vi "UHR-Fleezers Control (host) - 12.4.vi"() -> ()   [LabVIEW 2012] (continued)
          }
          frame #3 {
            n1108 = Wait (ms)(milliseconds to wait=u32 500) -> ()  [unwired: 1 out]
          }
          frame #4 {
            n1109 = property on="Confocal Image" class="Bool (strict)"("Val(Sgnl)"=TRUE ("Value (Signaling)")) -> ()  [unwired: 2 in, 2 out]
          }
          frame #5 {
            n1110 = Wait (ms)(milliseconds to wait=u32 2000) -> ()  [unwired: 1 out]
          }
          frame #6 {
            n1111 = while {
              stop <- w1611 stop-if-true
              n1112 = local read "Saving..."() -> (w1612:bool)
              n1113 = Not(x=w1612) -> (.not. x?=w1611:bool)
            }
          }
          frame #7 {
            n1114 = property on="Flip Green Filter" class="Bool (strict)"("Val(Sgnl)"=TRUE ("Value (Signaling)")) -> ()  [unwired: 2 in, 2 out]
            n1115 = property on="Green Laser ON" class="Bool (strict)"("Val(Sgnl)"=w1616) -> ()  [unwired: 2 in, 2 out]
            n1116 = property on="Laser interlacing mode" class="RadioBtnsControl (strict)"("Val(Sgnl)"=w1615) -> ()  [unwired: 2 in, 2 out]
          }
          frame #8 {
            n1117 = property on="Green FB On/Off" class="Bool (strict)"("Val(Sgnl)"=w1617) -> ()  [unwired: 2 in, 2 out]
          }
        }
      }
      event "Stop All": Value Change {
        n1118 = event-data() -> ()  [unwired: 1 in, 5 out]
        n1119 = local read "Delay (ms)"() -> (w1620:i32)
        n1120 = call "serial write macro.vi"("String"="l0", "Delay (ms)"=w1620, "VISA resource name"=w1623) -> ("read buffer"=w1618:string, "error out"=w1619:errorcluster, "VISA resource name out"=w1622:refnum<visa-resource-name>)
        n1121 = local write "read blue buffer"(w1618) -> ()
        n1122 = local write "Blue Error Out"(w1619) -> ()
        n1123 = VISA Close(VISA resource name=w1622) -> ()  [unwired: 1 in, 1 out]
        n1124 = local read "Stop All"() -> (w1624:bool)
      }
    }
    n1125 = node-c288() -> ()  [unwired: 1 in, 1 out]
  }
  n1126 = timed-loop "Basic control parameters (all FPGA settings, other basic controls)" {
    tunnel: w13 -> [w1633]
    shift-right: [w1632] -> _
    shift-left: errorcluster {"status"=FALSE, "code"=0, "source"=""} ("error out") -> [w1631]
    tunnel: [w1630] -> _
    timing: w127 -> [_]
    timing-out: [_] -> w126
    tunnel: w100 -> [w1629]
    tunnel: w72 -> [w1628]
    tunnel: w71 -> [w1627]
    tunnel: w70 -> [w1626]
    tunnel: w69 -> [w1625]
    stop <- w1630 stop-if-true
    n1127 = node-c288() -> ()  [unwired: 2 out]
    n1128 = event shown="[26] \"Invert APD Gate\", \"APD Gate ON Count\", \"APD Gate OFF Count\", \"APD Gate\", \"APD Integration Time (s)\", \"APD AO Scale Factor\", \"Duty Frequency (ON 1/N cycles)\", \"Interlace ON count\", \"Interlace OFF count\": Value Change" {
      selector: _ -> [_ _ _ _ _ _ _ _ _ _ _ _ _ _ _ _ _ _ _ _ _ _ _ _ _ _ _ _ _ _ _ _ _ _ _ _ _ _ _ _ _ _ _ _ _ _ _ _ _ _ _ _ _ _ _ _ _ _ _ _ _ _ _ _ _ _ _ _ _ _ _ _ _ _]
      dyn-events: _ -> [_ _ _ _ _ _ _ _ _ _ _ _ _ _ _ _ _ _ _ _ _ _ _ _ _ _ _ _ _ _ _ _ _ _ _ _ _ _ _ _ _ _ _ _ _ _ _ _ _ _ _ _ _ _ _ _ _ _ _ _ _ _ _ _ _ _ _ _ _ _ _ _ _ _]
      timeout: _ -> [_ _ _ _ _ _ _ _ _ _ _ _ _ _ _ _ _ _ _ _ _ _ _ _ _ _ _ _ _ _ _ _ _ _ _ _ _ _ _ _ _ _ _ _ _ _ _ _ _ _ _ _ _ _ _ _ _ _ _ _ _ _ _ _ _ _ _ _ _ _ _ _ _ _]
      tunnel: w1633 -> [w1674 _ _ _ w1712 _ w1734 _ _ _ _ w1800 _ _ w1843 w1849 w1856 w1861 w1952 _ w1968 w1993 w2014 w2035 w2056 w2085 w2111 w2114 w2118 w2213 w2218 w2256 _ w2291 w2295 w2306 w2310 w2314 _ w2322 _ _ _ _ _ _ _ _ _ _ _ _ _ _ _ _ _ w2700 _ w2717 _ w2724 w2742 _ w2749 w2757 w2772 w2788 w2794 _ w2803 _ w2822 _]
      tunnel: [w1673 _ _ _ w1702 _ w1733 _ _ w1765 _ w1779 _ _ w1842 w1845 w1855 w1858 w1946 _ w1967 w1992 w2012 w2033 w2054 w2079 w2109 _ w2116 w2211 w2216 w2254 _ w2289 w2293 w2297 w2308 w2312 _ w2320 _ _ _ _ _ _ _ _ _ _ _ _ _ _ _ _ _ w2698 _ _ _ _ w2739 _ _ _ _ _ _ _ _ _ _ _] -> w1632
      tunnel: w1631 -> [w1672 _ _ _ w1711 _ w1732 _ _ w1765 _ w1799 _ _ w1841 w1844 w1854 w1857 w1951 _ w1966 w1991 w2013 w2034 w2055 w2084 w2110 w2113 w2117 w2212 w2217 w2255 _ w2290 w2294 w2305 w2309 w2313 _ w2321 _ _ _ _ _ _ _ _ _ _ _ _ _ _ _ _ _ w2699 _ w2716 _ w2723 w2741 _ w2748 w2756 w2771 w2787 w2793 _ w2802 _ w2821 _]
      tunnel: [_ _ _ _ _ _ _ _ _ w1764 _ _ _ _ _ _ _ _ _ _ _ _ _ _ _ _ _ _ _ _ _ _ _ _ _ _ _ _ _ _ _ _ _ _ _ _ _ _ _ _ _ _ _ _ _ _ _ _ _ _ _ _ _ _ _ _ _ _ _ _ _ _ _ _] -> w1630
      tunnel: [_ _ _ _ _ _ _ "Round T1 X" _ _ _ _ _ _ _ _ _ _ _ _ _ _ _ _ _ _ _ _ _ _ _ _ _ _ _ _ _ _ _ _ _ _ _ _ _ _ _ _ _ _ _ _ _ _ _ _ _ _ _ _ _ _ _ _ _ _ _ _ _ _ _ _ _ _] -> _
      tunnel: [_ _ _ "Adjust Scale\nto Mean" _ _ _ _ _ _ _ _ _ _ _ _ _ _ _ _ _ _ _ _ _ _ _ _ "Test ttrig" _ _ _ _ _ _ _ _ _ _ _ _ _ _ _ _ _ _ "Flush Sample" "Flush Pump 3" "Flush Pump 1" "Clear Volume" _ _ _ _ _ _ _ _ _ _ _ _ _ _ _ _ _ _ _ _ _ _ _] -> _
      tunnel: [_ _ _ _ _ _ _ _ "Round T2 X" _ "Delayed Interlace Start" _ _ _ _ _ _ _ _ _ _ _ _ _ _ _ _ _ _ _ _ _ _ _ _ _ _ _ _ _ _ _ _ _ _ _ _ _ _ _ _ _ _ _ _ _ _ _ _ _ _ _ _ _ _ _ _ _ _ _ _ _ _ _] -> _
      tunnel: w1629 -> [_ _ _ _ _ _ _ _ _ _ _ _ _ _ _ _ _ _ _ _ _ _ _ _ _ _ _ _ _ _ _ _ _ _ _ _ _ _ _ _ _ _ _ w2479 w2486 w2493 w2498 w2507 _ _ w2613 _ _ _ _ _ _ _ _ _ _ _ _ _ _ _ _ _ _ _ _ _ _ _]
      tunnel: w1628 -> [_ _ _ _ _ _ _ _ _ _ _ _ _ _ _ _ _ _ _ _ _ _ _ _ _ _ _ _ _ _ _ _ _ _ _ _ _ _ _ _ _ w2396 _ _ _ _ _ _ w2551 _ _ w2619 _ w2628 _ w2642 _ _ _ _ _ _ _ _ _ _ _ _ _ _ _ _ _ _]
      tunnel: w1627 -> [_ _ _ _ _ _ _ _ _ _ _ _ _ _ _ _ _ _ _ _ _ _ _ _ _ _ _ _ _ _ _ _ _ _ _ _ _ _ _ _ _ _ _ _ _ _ _ _ _ _ _ _ _ _ _ _ _ _ _ _ _ _ _ _ _ _ _ _ _ _ _ _ _ _]
      tunnel: w1626 -> [_ _ _ _ _ _ _ _ _ _ _ _ _ _ _ _ _ _ _ _ _ _ _ _ _ _ _ _ _ _ _ _ _ _ _ _ _ _ _ _ w2333 _ _ _ _ _ _ _ _ w2581 _ _ w2624 _ w2635 _ w2667 _ _ _ _ _ _ _ _ _ _ _ _ _ _ _ _ _]
      tunnel: w1625 -> [_ _ _ _ _ _ _ _ _ _ _ _ _ _ _ _ _ _ _ _ _ _ _ _ _ _ _ _ _ _ _ _ _ _ _ _ _ _ _ _ _ _ _ _ _ _ _ _ _ _ _ _ _ _ _ _ _ _ _ _ _ _ _ _ _ _ _ _ _ _ _ _ _ _]
      event "AI Count (ticks)", "Sets to FIFO (Traps)", "Save ave N", "FPGA Ave.", "# Samples/channel", "N sets to save": Value Change {
        # "So that if 'Save ave N' is updated, the AOD scanning code updates too."
        n1129 = event-data() -> ()  [unwired: 6 out]
        n1130 = local read "AI Count (ticks)"() -> (w1656:u16)
        n1131 = Unbundle By Name("Sets to FIFO (Traps)") -> ("Set 1"=w1639:bool, "Set 2"=w1638:bool, "Set 3"=w1637:bool)
        n1132 = Boolean To (0,1)(Boolean="Sets to FIFO (Traps)") -> (0, 1=w1664:cluster{"Set 1":i16, "Set 2":i16, "Set 3":i16})
        n1133 = xnode "Read/Write Control"("FPGA VI Reference In"=w1674, "error in"=w1672, "ai count"=w1656, "Set 1"=w1639, "Set 2"=w1638, "Set 3"=w1637, "N of AI1 Int Acq Sets"="N Acq Sets (Traps + Fl.)") -> ("error out"=w1673:errorcluster)  [unwired: 1 out]
        n1134 = Cluster To Array(cluster=w1664) -> (array=w1663:i16[])
        n1135 = To Unsigned Long Integer(number=w1663) -> (unsigned 32bit integer=w1645:u32[])
        n1136 = local read "Scan steps (AOD)"() -> (w1665:u64)
        n1137 = Multiply(x=w1656, y="N Acq Sets (Traps + Fl.)") -> (x*y=w1654:u16)
        n1138 = Divide(x=40000000.0, y=w1656) -> (x/y=w1648:dbl)
        "AI rate (Hz)" <- w1648
        "Ave. Rate (Hz)" <- w1648
        n1139 = Add Array Elements(numeric array=w1645) -> (sum=w1657:u32)
        "Trap Sets" <- w1657
        n1140 = Reciprocal(x=w1648) -> (1/x=→"Ave. Period (s)":dbl)
        n1141 = property on="Scan steps (AOD)" class="DigNum (strict)"("Val(Sgnl)"=w1665) -> ()  [unwired: 2 in, 2 out]
        n1142 = Divide(x=w1648, y="N Acq Sets (Traps + Fl.)") -> (x/y=w1669:dbl)
        "Data Rate (Hz)" <- w1669
        n1143 = Reciprocal(x=w1669) -> (1/x=→"Data Period (s)":dbl)
        n1144 = local read "Save ave N"() -> (w1668:dbl)
        n1145 = Divide(x=w1669, y=w1668) -> (x/y=w1667:dbl)
        "Save Data Rate (Hz)" <- w1667
        n1146 = Reciprocal(x=w1667) -> (1/x=→"Save Data Period (s)":dbl)
        n1147 = Multiply(x=w1654, y="# Samples/trap") -> (x*y=w1652:u32)
        "Counts/DMA" <- w1652
        n1148 = property on="Trap Disp. Downsample" class="DigNum (strict)"("Maximum"="# Samples/trap") -> ()  [unwired: 2 in, 2 out]
        n1149 = Multiply(x=w1657, y="# Samples/trap") -> (x*y=w1646:u32)
        "# Samples/channel" <- w1646
        n1150 = Multiply(x=w1646, y=u32 8) -> (x*y=→"Trap AI Elements/DMA read":u32)
        n1151 = local read "APD Int. Count"() -> (w1653:u32)
        n1152 = Multiply(x=w1646, y=u32 3) -> (x*y=→"Trap Pos Elements/DMA read":u32)
        n1153 = Divide(x=w1652, y=w1653) -> (x/y=w1643:dbl)
        "APD Samples/FIFO Acq." <- w1643
        n1154 = Divide(x=w1652, y=40000000.0) -> (x/y=w1650:dbl)
        "DMA Update Period (s)" <- w1650
        n1155 = local read "Number of APDs"() -> (w1636:u8)
        n1156 = Multiply(x=w1636, y=w1643) -> (x*y=→"APD Elements/DMA read":dbl)
        n1157 = property on="APD Disp. Downsample" class="DigNum (strict)"("Maximum"=w1643) -> ()  [unwired: 2 in, 2 out]
        n1158 = local read "N sets to save"() -> (w1662:u32)
        n1159 = Multiply(x=w1650, y=w1662) -> (x*y=→"Total Time (s)":dbl)
        "FPGA Averaging" <- FALSE ("FPGA Averaging")
      }
      event "Remove Offset": Value Change {
        n1160 = event-data() -> ()  [unwired: 7 out]
        n1161 = local write "Remove Offset"(FALSE ("Remove Offset")) -> ()
        n1162 = local read "Bead Mean (nm)"() -> (w1676:dbl)
        n1163 = local read "Offset (nm)"() -> (w1677:dbl)
        n1164 = Add(x=w1676, y=w1677) -> (x+y=w1675:dbl)
        n1165 = local write "Offset (nm)"(w1675) -> ()
        n1166 = disable-structure shown="Disabled" {
          frame Disabled {
            n1167 = local read "Bead Mean (nm)"() -> (w1682:dbl)
            n1168 = Add(y=w1682) -> (x=w1681:dbl, x+y=w1680:dbl)
            n1169 = Subtract(x=w1682, y=w1681) -> (x-y=w1679:dbl)
            n1170 = property on="Bead Separation" class="WFChart (strict)"("YScale.Minimum"=w1679) -> ()  [unwired: 2 in, 2 out]
            n1171 = property on="Bead Separation" class="WFChart (strict)"("YScale.Maximum"=w1680) -> ()  [unwired: 2 in, 2 out]
          }
          frame Enabled {
          }
        }
      }
      event "Detector Type": Value Change {
        n1172 = event-data() -> ()  [unwired: 7 out]
        n1173 = local read "AI labels"() -> (w1683:string[])
        n1174 = property on="High Res. Display" class="Ring (strict)"("Strings []"=w1683) -> ()  [unwired: 2 in, 2 out]
        n1175 = Build Array (concatenate)(w1683, "none") -> (w1684:string[])
        n1176 = property on="FFT 1 Choice 1" class="Ring (strict)"("Strings []"=w1684) -> ()  [unwired: 2 in, 2 out]
        n1177 = property on="FFT 1 Choice 2" class="Ring (strict)"("Strings []"=w1684) -> ()  [unwired: 2 in, 2 out]
        n1178 = property on="FFT 2 Choice 1" class="Ring (strict)"("Strings []"=w1684) -> ()  [unwired: 2 in, 2 out]
        n1179 = property on="FFT 2 Choice 2" class="Ring (strict)"("Strings []"=w1684) -> ()  [unwired: 2 in, 2 out]
        n1180 = Bundle("APD 1", "APD 2") -> (w1687:cluster{string, string})  [unwired: 1 out]
        n1181 = Cluster To Array(cluster=w1687) -> (array=w1685:string[])
        n1182 = Build Array (concatenate)(w1685, w1684) -> (w1689:string[])
        n1183 = Array Size(array=w1689) -> (size(s)=w1690:i32)
        n1184 = property on="Signals to Plot" class="LstBox (strict)"("Item Names"=w1689) -> ()  [unwired: 2 in, 2 out]
        n1185 = property on="Signals to Plot" class="LstBox (strict)"("Number of Rows"=w1690) -> ()  [unwired: 2 in, 2 out]
        n1186 = property on="All Signals" class="WFChart (strict)"("LegNumRows"=w1690) -> ()  [unwired: 2 in, 2 out]
      }
      event "Adjust Scale\nto Mean": Value Change {
        n1187 = event-data() -> ()  [unwired: 7 out]
        n1188 = local read "APD 1 Rate (Hz)"() -> (w1699:dbl)
        n1189 = Multiply(x=1000.0, y="Above (kHz)") -> (x*y=w1697:dbl)
        n1190 = Multiply(x=1000.0, y="Below (kHz)") -> (x*y=w1695:dbl)
        n1191 = Add(x=w1697, y=w1699) -> (x+y=w1692:dbl)
        n1192 = Subtract(x=w1699, y=w1695) -> (x-y=w1693:dbl)
        n1193 = property on="APD Chart" class="WFChart (strict)"("YScale.Minimum"=w1693) -> ()  [unwired: 2 in, 2 out]
        n1194 = property on="APD Chart" class="WFChart (strict)"("YScale.Maximum"=w1692) -> ()  [unwired: 2 in, 2 out]
      }
      event "Phase adj. (AI1)", "+ phase (AI1)", "- phase (AI1)": Value Change {
        n1195 = event-data() -> ()  [unwired: 7 out]
        n1196 = Negate(x="Phase adj. (AI1)") -> (-x=w1709:i16)
        n1197 = Select(t=w1709, s="- phase (AI1)", f="Phase adj. (AI1)") -> (s? t:f=w1708:i16)
        n1198 = xnode "Read/Write Control"("FPGA VI Reference In"=w1712, "error in"=w1711, "Phase count adjustment"=w1708) -> ("FPGA VI Reference Out"=w1707:T19, "error out"=w1706:errorcluster)
        n1199 = Or(x="- phase (AI1)", y="+ phase (AI1)") -> (x .or. y?=w1703:bool)
        n1200 = xnode "Read/Write Control"("FPGA VI Reference In"=w1707, "error in"=w1706, "+ phase"=w1703) -> ("error out"=w1702:errorcluster)  [unwired: 1 out]
      }
      event "Signals to Plot": Double Click {
        w1715 = u32 9868950 ("Color Box")
        n1201 = event-data() -> ("Row"=w1717:i32)  [unwired: 9 out]
        n1202 = property on="All Signals" class="WFChart (strict)"("Active Plot"=w1717) -> (error out=w1728:errorcluster)  [unwired: 2 in, 1 out]
        n1203 = property on="All Signals" class="WFChart (strict)" props=["Plot", "Visible?", "Plot", "Plot Color"](error in=w1728) -> (error out=w1727:errorcluster, "Plot.Visible?"=w1726:bool)  [unwired: 1 in, 2 out]
        n1204 = Select(t=FALSE ("Plot.Visible"), s=w1726, f=TRUE ("Plot.Visible")) -> (s? t:f=w1721:bool)
        n1205 = property on="All Signals" class="WFChart (strict)"(error in=w1727, "Plot.Visible?"=w1721) -> (error out=w1723:errorcluster)  [unwired: 1 in, 1 out]
        n1206 = property on="All Signals" class="WFChart (strict)"(error in=w1723) -> (error out=w1718:errorcluster, "Plot.Plot Color"=w1722:u32)  [unwired: 1 in, 1 out]
        n1207 = property on="Signals to Plot" class="LstBox (strict)"(error in=w1718, "Active Row"=w1717) -> (error out=w1716:errorcluster)  [unwired: 1 in, 1 out]
        n1208 = Select(t=w1722, s=w1721, f=u32 0) -> (s? t:f=w1719:u32)
        n1209 = property on="Signals to Plot" class="LstBox (strict)"(error in=w1716, "CellFontColor"=w1719, "SelColor"=w1715, "CellBG"=w1715, "CellFontSize"=u32 20 ("Active Row:Cell Font:Size"), "CellFontBold"=TRUE ("Active Row:Cell Font:Bold")) -> ()  [unwired: 1 in, 2 out]
      }
      event "BD 1 Frequency 1 (MHz)", "BD 1 Frequency 2 (MHz)", "BD 1 Frequency 3 (MHz)", "BD 2 Frequency 1 (MHz)", "BD 2 Frequency 2 (MHz)", "BD 2 Frequency 3 (MHz)", "Trap Delta (MHz)": Value Change {
        n1210 = event-data() -> ("CtlRef"=w1731:refnum<vi>)  [unwired: 6 out]
        n1211 = control-ref of="Trap Delta (MHz)"() -> (w1730:refnum<vi>)
        n1212 = Equal?(x=w1730, y=w1731) -> (x = y?=w1729:bool)
        n1213 = case shown="False" "Oscillate Set 1" {
          tunnel: w1734 -> [w1754 _]
          tunnel: [w1753 w1757] -> w1733
          tunnel: w1732 -> [w1752 w1757]
          tunnel: w1729 -> [w1737 _]
          frame False {
            n1214 = local read "BD 1 Frequency 2 (MHz)"() -> (w1741:dbl)
            n1215 = local read "BD 1 Frequency 1 (MHz)"() -> (w1739:dbl)
            n1216 = Subtract(x=w1741, y="Trap Delta (MHz)") -> (x-y=w1738:dbl)
            n1217 = Select(t=w1738, s=w1737, f=w1739) -> (s? t:f=w1736:dbl)
            n1218 = local read "Y RF Frequency Limits (MHz)"() -> (w1742:T16)
            n1219 = local read "X RF Frequency Limits (MHz)"() -> (w1743:T16)
            n1220 = local read "BD 1 Frequency 3 (MHz)"() -> (w1755:dbl)
            n1221 = local write "BD 1 Frequency 1 (MHz)"(w1736) -> ()
            n1222 = local read "BD 2 Frequency 1 (MHz)"() -> (w1746:dbl)
            n1223 = local read "BD 2 Frequency 2 (MHz)"() -> (w1745:dbl)
            n1224 = local read "BD 2 Frequency 3 (MHz)"() -> (w1756:dbl)
            n1225 = call "set RF board frequency - interlace.vi"("Board 2 Frequency Limits"=w1742, "Board 1 Frequency Limits"=w1743, "error in"=w1752, "FPGA VI Reference In"=w1754, "Board 2 Frequency 3 (MHz)"=w1756, "Board 1 Frequency 3 (MHz)"=w1755, "Board 2 Frequency 2 (MHz)"=w1745, "Board 2 Frequency 1 (MHz)"=w1746, "Board 1 Frequency 2 (MHz)"=w1741, "Board 1 Frequency 1  (MHz)"=w1736) -> ("error out"=w1753:errorcluster)  [unwired: 1 out]
            n1226 = Subtract(x=w1746, y=w1745) -> (x-y=w1750:dbl)
            n1227 = Subtract(x=w1736, y=w1741) -> (x-y=w1751:dbl)
            n1228 = Square(x=w1750) -> (x^2=w1748:dbl)
            n1229 = Square(x=w1751) -> (x^2=w1749:dbl)
            n1230 = Add(x=w1749, y=w1748) -> (x+y=w1747:dbl)
            n1231 = Square Root(x=w1747) -> (sqrt(x)=w1744:dbl)
            n1232 = local write "Trap Delta (MHz)"(w1744) -> ()
            n1233 = property on="Initial delta (MHz)" class="DigNum (strict)"("Val(Sgnl)"=w1744) -> ()  [unwired: 2 in, 2 out]
          }
          frame True {
          }
        }
      }
      event "Round T1 X": Value Change {
        n1234 = event-data() -> ()  [unwired: 7 out]
        n1235 = local read "BD 1 Frequency 1 (MHz)"() -> (w1760:dbl)
        n1236 = Round To Nearest(number=w1760) -> (nearest integer value=w1759:dbl)
        n1237 = property on="BD 1 Frequency 1 (MHz)" class="DigNum (strict)"("Val(Sgnl)"=w1759) -> ()  [unwired: 2 in, 2 out]
      }
      event "Round T2 X": Value Change {
        n1238 = event-data() -> ()  [unwired: 7 out]
        n1239 = local read "BD 1 Frequency 2 (MHz)"() -> (w1762:dbl)
        n1240 = Round To Nearest(number=w1762) -> (nearest integer value=w1761:dbl)
        n1241 = property on="BD 1 Frequency 2 (MHz)" class="DigNum (strict)"("Val(Sgnl)"=w1761) -> ()  [unwired: 2 in, 2 out]
      }
      event "Stop All": Value Change {
        n1242 = event-data() -> ()  [unwired: 7 out]
        n1243 = local read "Stop All"() -> (w1764:bool)
      }
      event "Delayed Interlace Start": Value Change {
        n1244 = event-data() -> ()  [unwired: 7 out]
        n1245 = flat-sequence {
          frame #0 {
            n1246 = Multiply(x="Delay to Interlace (s)", y=1000.0) -> (x*y=w1767:dbl)
            n1247 = Wait (ms)(milliseconds to wait=w1767) -> ()  [unwired: 1 out]
          }
          frame #1 {
            n1248 = property on="Laser interlacing mode" class="RadioBtnsControl (strict)"("Val(Sgnl)"=enum32{"Laser ON", "Laser OFF", "Interlace"}."Interlace" ("Value (Signaling)")) -> ()  [unwired: 2 in, 2 out]
          }
        }
      }
      event "BD 1 Amplitude 1 (%)", "BD 1 Amplitude 2 (%)", "BD 1 Amplitude 3 (%)", "BD 2 Amplitude 1 (%)", "BD 2 Amplitude 2 (%)", "BD 2 Amplitude 3 (%)", "Trap 1 ON", "Trap 2 ON", "Trap 3 ON", "Feedback On/Off", "All FB On/Off": Value Change {
        w1791 = i16 1 ("f")
        n1249 = event-data() -> ()  [unwired: 7 out]
        n1250 = local write "Trap 1 (ON/OFF)"("Trap 1 ON") -> ()
        n1251 = local write "Trap 2 (ON/OFF)"("Trap 2 ON") -> ()
        n1252 = Boolean To (0,1)(Boolean="Trap 3 ON") -> (0, 1=w1792:i16)
        n1253 = Boolean To (0,1)(Boolean="Trap 1 ON") -> (0, 1=w1793:i16)
        n1254 = Boolean To (0,1)(Boolean="Trap 2 ON") -> (0, 1=w1794:i16)
        n1255 = Select(t=w1794, s="Trap ON/OFF X or Y Amp?", f=w1791) -> (s? t:f=w1789:i16)
        n1256 = Select(t=w1793, s="Trap ON/OFF X or Y Amp?", f=w1791) -> (s? t:f=w1790:i16)
        n1257 = Select(t=w1792, s="Trap ON/OFF X or Y Amp?", f=w1791) -> (s? t:f=w1788:i16)
        n1258 = Select(t=w1791, s="Trap ON/OFF X or Y Amp?", f=w1794) -> (s? t:f=w1786:i16)
        n1259 = Select(t=w1791, s="Trap ON/OFF X or Y Amp?", f=w1793) -> (s? t:f=w1787:i16)
        n1260 = Select(t=w1791, s="Trap ON/OFF X or Y Amp?", f=w1792) -> (s? t:f=w1785:i16)
        n1261 = And(x="All FB On/Off", y="Feedback On/Off") -> (x .and. y?=w1783:cluster{"Set 1":bool, "Set 2":bool})
        n1262 = local read "BD 1 Amplitude 1 (%)"() -> (w1803:dbl)
        n1263 = local read "BD 1 Amplitude 2 (%)"() -> (w1802:dbl)
        n1264 = local read "BD 1 Amplitude 3 (%)"() -> (w1801:dbl)
        n1265 = Unbundle By Name(w1783) -> ("Set 1"=w1778:bool, "Set 2"=w1775:bool)
        n1266 = local read "Y RF Amplitude Limits (%)"() -> (w1771:T16)
        n1267 = local read "X RF Amplitude Limits (%)"() -> (w1772:T16)
        n1268 = local read "BD 2 Amplitude 1 (%)"() -> (w1804:dbl)
        n1269 = local read "BD 2 Amplitude 2 (%)"() -> (w1805:dbl)
        n1270 = local read "BD 2 Amplitude 3 (%)"() -> (w1806:dbl)
        n1271 = And(x="Trap 2 ON", y=w1775) -> (x .and. y?=w1773:bool)
        n1272 = And(x="Trap 1 ON", y=w1778) -> (x .and. y?=w1776:bool)
        n1273 = Multiply(x=w1790, y=w1803) -> (x*y=w1798:dbl)
        n1274 = Multiply(x=w1802, y=w1789) -> (x*y=w1796:dbl)
        n1275 = Multiply(x=w1801, y=w1788) -> (x*y=w1797:dbl)
        n1276 = Multiply(x=w1804, y=w1787) -> (x*y=w1807:dbl)
        n1277 = Multiply(x=w1805, y=w1786) -> (x*y=w1808:dbl)
        n1278 = Multiply(x=w1806, y=w1785) -> (x*y=w1809:dbl)
        n1279 = call "set RF board amplitude - interlace.vi"("Board 2 Amplitude Limits"=w1771, "Board 1 Amplitude Limits"=w1772, "error in"=w1799, "FPGA VI Reference In"=w1800, "Board 2 Amplitude 3 (%)"=w1809, "Board 1 Amplitude 3 (%)"=w1797, "Board 2 Amplitude 2 (%)"=w1808, "Board 2 Amplitude 1 (%)"=w1807, "Board 1 Amplitude 2 (%)"=w1796, "Board 1 Amplitude 1 (%)"=w1798) -> ("error out"=w1780:errorcluster, "FPGA VI Reference Out"=w1781:T19)
        n1280 = xnode "Read/Write Control"("FPGA VI Reference In"=w1781, "error in"=w1780, "FB On/Off Set 1"=w1776, "FB On/Off Set 2"=w1773) -> ("error out"=w1779:errorcluster)  [unwired: 1 out]
      }
      event "Load parameters": Value Change {
        n1281 = event-data() -> ()  [unwired: 7 out]
        n1282 = property on="Saved AOD Raster Scan Parameter Sets" class="Arr (strict)"() -> ("Index Values"=w1820:u32[])  [unwired: 2 in, 2 out]
        n1283 = Index Array(array=w1820, index=0) -> (element=w1817:u32)
        n1284 = local write "Load parameters"(FALSE ("Load parameters")) -> ()
        n1285 = Index Array(array="Saved AOD Raster Scan Parameter Sets", index=w1817) -> (element=w1816:T28)
        n1286 = Unbundle By Name(w1816) -> ("Scan Range AOD (nm) 2"=w1815:dbl, "Step Size AOD (nm) 2"=w1814:dbl, "Scan Speed AOD (nm/s) 2"=w1813:dbl, "Number of scans (AOD) 2"=w1812:u16)
        n1287 = flat-sequence {
          tunnel: w1815 -> [w1823]
          tunnel: w1814 -> [w1822]
          tunnel: w1813 -> [w1821]
          tunnel: w1812 -> [w1824]
          frame #0 {
            n1288 = local write "Scan Speed (nm/s)"(w1821) -> ()
            n1289 = local write "Scan Range (nm)"(w1823) -> ()
            n1290 = local write "Step Size (nm)"(w1822) -> ()
          }
          frame #1 {
            n1291 = property on="Number of F/B Scans (AOD)" class="DigNum (strict)"("Val(Sgnl)"=w1824) -> ()  [unwired: 2 in, 2 out]
          }
        }
      }
      event "Trap 1 (ON/OFF)", "Trap 2 (ON/OFF)": Value Change {
        n1292 = event-data() -> ()  [unwired: 7 out]
        n1293 = property on="Trap 2 ON" class="Bool (strict)"("Val(Sgnl)"="Trap 2 (ON/OFF)") -> ()  [unwired: 2 in, 2 out]
        n1294 = property on="Trap 1 ON" class="Bool (strict)"("Val(Sgnl)"="Trap 1 (ON/OFF)") -> ()  [unwired: 2 in, 2 out]
      }
      event "DIO count 1 (ticks)", "DIO count 2 (ticks)", "DIO count 3 (ticks)", "Interlace", "Number Interlace Sets", "Not-Interlacing Set": Value Change {
        n1295 = event-data() -> ()  [unwired: 7 out]
        n1296 = local read "DIO count 3 (ticks)"() -> (w1837:u16)
        n1297 = local read "DIO count 1 (ticks)"() -> (w1839:u16)
        n1298 = local read "DIO count 2 (ticks)"() -> (w1838:u16)
        n1299 = To Unsigned Byte Integer(number="Not-Interlacing Set") -> (unsigned 8bit integer=w1828:u8)
        n1300 = Add(x=w1828, y=u8 1) -> (x+y=w1832:u8)
        n1301 = xnode "Read/Write Control"("FPGA VI Reference In"=w1843, "error in"=w1841, "DIO count 1 (ticks)"=w1839, "DIO count 2 (ticks)"=w1838, "DIO count 3 (ticks)"=w1837, "Interlace ON/OFF"="Interlace", "Number Interlace Cycles"="Number Interlace Sets", "Interlace Off Parameters"=w1832) -> ("error out"=w1842:errorcluster)  [unwired: 1 out]
        n1302 = Build Array(w1839, w1838, w1837) -> (w1830:u16[])
        n1303 = Split 1D Array(array=w1830, index="Number Interlace Sets") -> (first subarray=w1840:u16[])  [unwired: 1 out]
        n1304 = Index Array(array=w1830, index=w1828) -> (element=w1829:u16)
        n1305 = Add Array Elements(numeric array=w1840) -> (sum=w1834:u16)
        n1306 = Select(t=w1834, s="Interlace", f=w1829) -> (s? t:f=→"Total Counts (ticks)":u16)
      }
      event "Reset Feedback": Value Change {
        n1307 = event-data() -> ()  [unwired: 7 out]
        n1308 = Unbundle By Name("Reset Feedback") -> ("Set 1"=w1847:bool, "Set 2"=w1846:bool)
        n1309 = xnode "Read/Write Control"("FPGA VI Reference In"=w1849, "error in"=w1844, "FB Reset Set 1"=w1847, "FB Reset Set 2"=w1846) -> ("error out"=w1845:errorcluster)  [unwired: 1 out]
      }
      event "Trap Intensity PID Gains": Value Change {
        n1310 = event-data() -> ()  [unwired: 7 out]
        n1311 = Unbundle By Name("Trap Intensity PID Gains") -> ("proportional gain (Kc)"=w1852:i16, "integral gain (Kc*Ts/Ti)"=w1851:i16, "derivative gain (Kc*Td/Ts)"=w1850:i16)
        n1312 = xnode "Read/Write Control"("FPGA VI Reference In"=w1856, "error in"=w1854, "P1"=w1852, "I1"=w1851, "D1"=w1850) -> ("error out"=w1855:errorcluster)  [unwired: 1 out]
      }
      event "AI2 to Setpoint", "Setpoints (V)": Value Change {
        n1313 = event-data() -> ()  [unwired: 7 out]
        n1314 = xnode "Read/Write Control"("FPGA VI Reference In"=w1861, "error in"=w1857) -> ("FPGA VI Reference Out"=w1860:T19, "error out"=w1859:errorcluster, "AI2 Y Sum Set 1"=w1868:i16, "AI2 Y Sum Set 2"=w1867:i16)
        n1315 = Cluster To Array(cluster="AI2 to Setpoint") -> (array=w1871:bool[])
        n1316 = local read "AI2 (V)"() -> (w1869:cluster{"Set 1":dbl, "Set 2":dbl})
        n1317 = Or Array Elements(Boolean array=w1871) -> (logical OR=w1872:bool)
        n1318 = Bundle By Name(cluster=w1869, "Set 1"=w1868, "Set 2"=w1867) -> (w1866:cluster{"Set 1":dbl, "Set 2":dbl})
        n1319 = Divide(x=w1866, y=3276.7) -> (x/y=w1865:cluster{"Set 1":dbl, "Set 2":dbl})
        "AI2 (V)" <- w1865
        n1320 = case shown="True" w1872 {
          tunnel: [w1875 w1892] -> w1864
          tunnel: "AI2 to Setpoint" -> [_ w1888]
          tunnel: "Setpoints (V)" -> [w1876 w1891]
          tunnel: w1865 -> [_ w1885]
          frame False {
            n1321 = Multiply(x=3276.7, y=w1876) -> (x*y=w1877:cluster{"Set 1":dbl, "Set 2":dbl})
            n1322 = To Word Integer(number=w1877) -> (16bit integer=w1875:cluster{"Set 1":i16, "Set 2":i16})
          }
          frame True {
            n1323 = Unbundle By Name(w1885) -> ("Set 1"=w1884:dbl, "Set 2"=w1883:dbl)
            n1324 = Unbundle By Name(w1891) -> ("Set 1"=w1890:dbl, "Set 2"=w1889:dbl)
            n1325 = Unbundle By Name(w1888) -> ("Set 1"=w1887:bool, "Set 2"=w1886:bool)
            n1326 = Select(t=w1884, s=w1887, f=w1890) -> (s? t:f=w1882:dbl)
            n1327 = Select(t=w1883, s=w1886, f=w1889) -> (s? t:f=w1881:dbl)
            n1328 = Bundle By Name(cluster=w1891, "Set 1"=w1882, "Set 2"=w1881) -> (w1879:cluster{"Set 1":dbl, "Set 2":dbl})
            n1329 = local write "Setpoints (V)"(w1879) -> ()
            n1330 = Multiply(x=3276.7, y=w1879) -> (x*y=w1880:cluster{"Set 1":dbl, "Set 2":dbl})
            n1331 = To Word Integer(number=w1880) -> (16bit integer=w1892:cluster{"Set 1":i16, "Set 2":i16})
          }
        }
        n1332 = Unbundle By Name(w1864) -> ("Set 1"=w1863:i16, "Set 2"=w1862:i16)
        n1333 = xnode "Read/Write Control"("FPGA VI Reference In"=w1860, "error in"=w1859, "FB Setpoint Set 1"=w1863, "FB Setpoint Set 2"=w1862) -> ("error out"=w1858:errorcluster)  [unwired: 1 out]
      }
      event "+ phase (GI)", "- phase (GI)", "+ phase (GI) 2", "- phase (GI) 2", "+ phase (RI)", "- phase (RI)", "+ phase (RI) 2", "- phase (RI) 2", "+ phase (Green FB)", "- phase (Green FB)", "+ phase (RI FB)", "- phase (RI FB)": Value Change {
        n1334 = event-data() -> ()  [unwired: 7 out]
        n1335 = Or(x="+ phase (GI)", y="- phase (GI)") -> (x .or. y?=w1945:bool)
        n1336 = Negate(x="Phase adj. (GI)") -> (-x=w1950:i16)
        n1337 = Select(t=w1950, s="+ phase (GI)", f="Phase adj. (GI)") -> (s? t:f=w1949:i16)
        n1338 = Or(x="+ phase (GI) 2", y="- phase (GI) 2") -> (x .or. y?=w1936:bool)
        n1339 = Negate(x="Phase adj. (GI) 2") -> (-x=w1941:i16)
        n1340 = Select(t=w1941, s="+ phase (GI) 2", f="Phase adj. (GI) 2") -> (s? t:f=w1937:i16)
        n1341 = Negate(x="Phase adj. (RI)") -> (-x=w1935:i16)
        n1342 = Or(x="+ phase (RI)", y="- phase (RI)") -> (x .or. y?=w1931:bool)
        n1343 = Select(t=w1935, s="+ phase (RI)", f="Phase adj. (RI)") -> (s? t:f=w1930:i16)
        n1344 = Negate(x="Phase adj. (RI) 2") -> (-x=w1929:i16)
        n1345 = Or(x="+ phase (RI) 2", y="- phase (RI) 2") -> (x .or. y?=w1918:bool)
        n1346 = Select(t=w1929, s="+ phase (RI) 2", f="Phase adj. (RI) 2") -> (s? t:f=w1925:i16)
        n1347 = Or(x="+ phase (Green FB)", y="- phase (Green FB)") -> (x .or. y?=w1919:bool)
        n1348 = Negate(x="Phase adj. (Green FB)") -> (-x=w1924:i16)
        n1349 = Select(t=w1924, s="+ phase (Green FB)", f="Phase adj. (Green FB)") -> (s? t:f=w1920:i16)
        n1350 = Or(x="+ phase (RI FB)", y="- phase (RI FB)") -> (x .or. y?=w1912:bool)
        n1351 = Negate(x="Phase adj. (RI FB)") -> (-x=w1917:i16)
        n1352 = Select(t=w1917, s="+ phase (RI FB)", f="Phase adj. (RI FB)") -> (s? t:f=w1913:i16)
        n1353 = Negate(x="Phase adj. (BI AO)") -> (-x=w1911:i16)
        n1354 = Or(x="+ phase (BI AO)", y="- phase (BI AO)") -> (x .or. y?=w1896:bool)
        n1355 = Select(t=w1911, s="+ phase (BI AO)", f="Phase adj. (BI AO)") -> (s? t:f=w1899:i16)
        n1356 = Negate(x="Phase adj. (BI DO)") -> (-x=w1907:i16)
        n1357 = Or(x="+ phase (BI DO)", y="- phase (BI DO)") -> (x .or. y?=w1895:bool)
        n1358 = Select(t=w1907, s="+ phase (BI DO)", f="Phase adj. (BI DO)") -> (s? t:f=w1898:i16)
        n1359 = Negate(x="Phase adj. (BI AI)") -> (-x=w1903:i16)
        n1360 = Or(x="+ phase (BI AI)", y="- phase (BI AI)") -> (x .or. y?=w1894:bool)
        n1361 = Select(t=w1903, s="+ phase (BI AI)", f="Phase adj. (BI AI)") -> (s? t:f=w1897:i16)
        n1362 = xnode "Read/Write Control"("FPGA VI Reference In"=w1952, "error in"=w1951, "Phase count adjustment (GI)"=w1949, "Phase count adjustment (GI) 2"=w1937, "Phase count adjustment (RI)"=w1930, "Phase count adjustment (RI) 2"=w1925, "Phase count adjustment (Green FB)"=w1920, "Phase count adjustment (Red FB)"=w1913, "Phase count adjustment (BI AO)"=w1899, "Phase count adjustment (BI D)"=w1898, "Phase count adjustment (Blue Int)"=w1897) -> ("FPGA VI Reference Out"=w1947:T19, "error out"=w1948:errorcluster)
        n1363 = xnode "Read/Write Control"("FPGA VI Reference In"=w1947, "error in"=w1948, "+ phase (GI)"=w1945, "+ phase (GI) 2"=w1936, "+ phase (RI)"=w1931, "+ phase (RI) 2"=w1918, "+ phase (Green FB)"=w1919, "+ phase (Red FB)"=w1912, "+ phase (BI AO)"=w1896, "+ phase (BI D)"=w1895, "+ phase (Blue Int)"=w1894) -> ("error out"=w1946:errorcluster)  [unwired: 1 out]
      }
      event "Green Laser ON/OFF", "Red Laser ON/OFF", "Blue Laser ON/OFF": Value Change {
        # "This loop shouldn't be initialized.  The main 'laser ON' settings should dominate and set the others."
        n1364 = event-data() -> ()  [unwired: 7 out]
        n1365 = property on="Red Laser ON" class="Bool (strict)"("Val(Sgnl)"="Red Laser ON/OFF") -> ()  [unwired: 2 in, 2 out]
        n1366 = property on="Blue Laser ON" class="Bool (strict)"("Val(Sgnl)"="Blue Laser ON/OFF") -> ()  [unwired: 2 in, 2 out]
        n1367 = property on="Green Laser ON" class="Bool (strict)"("Val(Sgnl)"="Green Laser ON/OFF") -> ()  [unwired: 2 in, 2 out]
      }
      event "Laser interlacing mode", "Green Laser ON", "Red Laser ON", "Blue Laser ON": Value Change {
        n1368 = event-data() -> ()  [unwired: 7 out]
        n1369 = local write "Green Laser ON/OFF"("Green Laser ON") -> ()
        n1370 = local write "Blue Laser ON/OFF"("Blue Laser ON") -> ()
        n1371 = local write "Red Laser ON/OFF"("Red Laser ON") -> ()
        n1372 = case shown="True" "Green Laser ON" {
          tunnel: "Laser interlacing mode" -> [_ w1989]
          tunnel: [enum32{"Laser ON", "Laser OFF", "Interlace"}."Laser OFF" ("Green laser mode") w1989] -> w1965
          tunnel: [FALSE w1985] -> w1964
          frame False {
          }
          frame True {
            n1373 = local read "Green FB On/Off"() -> (w1986:bool)
            n1374 = Equal?(x=w1989, y=enum32{"Laser ON", "Laser OFF", "Interlace"}."Interlace") -> (x = y?=w1987:bool)
            n1375 = And(x=w1987, y=w1986) -> (x .and. y?=w1985:bool)
          }
        }
        n1376 = case shown="True" "Red Laser ON" {
          tunnel: "Laser interlacing mode" -> [_ w1982]
          tunnel: [enum32{"Laser ON", "Laser OFF", "Interlace"}."Laser OFF" ("Green laser mode") w1982] -> w1961
          tunnel: [FALSE w1978] -> w1960
          frame False {
          }
          frame True {
            n1377 = local read "Red FB On/Off"() -> (w1979:bool)
            n1378 = Equal?(x=w1982, y=enum32{"Laser ON", "Laser OFF", "Interlace"}."Interlace") -> (x = y?=w1980:bool)
            n1379 = And(x=w1980, y=w1979) -> (x .and. y?=w1978:bool)
          }
        }
        n1380 = case shown="True" "Blue Laser ON" {
          tunnel: "Laser interlacing mode" -> [_ w1973]
          tunnel: [enum32{"Laser ON", "Laser OFF", "Interlace"}."Laser OFF" ("Green laser mode") w1973] -> w1957
          tunnel: [FALSE w1971] -> w1956
          frame False {
          }
          frame True {
            n1381 = local read "Blue FB On/Off"() -> (w1972:bool)
            n1382 = Equal?(x=w1973, y=enum32{"Laser ON", "Laser OFF", "Interlace"}."Interlace") -> (x = y?=w1974:bool)
            n1383 = And(x=w1974, y=w1972) -> (x .and. y?=w1971:bool)
          }
        }
        n1384 = xnode "Read/Write Control"("FPGA VI Reference In"=w1968, "error in"=w1966, "Operating Mode"=w1965, "Operating Mode 2"=w1965, "Green FB On/Off"=w1964, "Red Laser Operating Mode"=w1961, "RI Operating Mode 2"=w1961, "Red FB On/Off"=w1960, "BI Operating Mode (AO)"=w1957, "Blue Laser Operating Mode (D)"=w1957, "Blue FB On/Off"=w1956) -> ("error out"=w1967:errorcluster)  [unwired: 1 out]
      }
      event "Invert laser interlacing": Value Change {
        n1385 = event-data() -> ()  [unwired: 7 out]
        n1386 = xnode "Read/Write Control"("FPGA VI Reference In"=w1993, "error in"=w1991, "Invert GI"="Invert laser interlacing", "Invert GI 2"="Invert laser interlacing", "Invert RI"="Invert laser interlacing", "Invert RI 2"="Invert laser interlacing", "Invert BI (AO)"="Invert laser interlacing", "Invert BI (D)"="Invert laser interlacing") -> ("error out"=w1992:errorcluster)  [unwired: 1 out]
      }
      event "Green FB Setpoint (mV)", "Green FB Gains", "Green FB On/Off", "Green Intensity % (FB OFF)", "Green int current ON count adj": Value Change {
        n1387 = event-data() -> ()  [unwired: 7 out]
        n1388 = local read "Green FB Setpoint (mV)"() -> (w2004:dbl)
        n1389 = Multiply(x=w2004, y=3.2767) -> (x*y=w2003:dbl)
        n1390 = local read "Green Intensity % (FB OFF)"() -> (w2007:dbl)
        n1391 = Multiply(x=w2007, y=655.35) -> (x*y=w2008:dbl)
        n1392 = To Unsigned Word Integer(number=w2008) -> (unsigned 16bit integer=w2006:u16)
        n1393 = local read "Green int current ON count adj"() -> (w2010:u32)
        n1394 = local read "Laser interlacing mode"() -> (w2000:enum32{"Laser ON", "Laser OFF", "Interlace"})
        n1395 = local read "Green FB Gains"() -> (w1997:T9)
        n1396 = local read "Green Laser ON"() -> (w2001:bool)
        n1397 = local read "Green FB On/Off"() -> (w2011:bool)
        n1398 = Equal?(x=w2000, y=enum32{"Laser ON", "Laser OFF", "Interlace"}."Interlace") -> (x = y?=w1998:bool)
        n1399 = Unbundle By Name(w1997) -> ("proportional gain (Kc)"=w1996:i16, "integral gain (Kc*Ts/Ti)"=w1995:i16, "derivative gain (Kc*Td/Ts)"=w1994:i16)
        n1400 = Compound Arithmetic op=AND(w1998, w2011, w2001) -> (w2002:bool)
        n1401 = xnode "Read/Write Control"("FPGA VI Reference In"=w2014, "error in"=w2013, "Green FB Setpoint"=w2003, "Green FB On/Off"=w2002, "Current Out"=w2006, "Green int current ON count adj"=w2010, "P3"=w1996, "I3"=w1995, "D3"=w1994) -> ("error out"=w2012:errorcluster)  [unwired: 1 out]
      }
      event "Blue FB Setpoint (mV)", "Blue FB Gains", "Blue FB On/Off", "Blue Intensity % (FB OFF)", "Blue int AO ON count adjust": Value Change {
        # "16 bit analog out"
        n1402 = event-data() -> ()  [unwired: 7 out]
        n1403 = Multiply(x="Blue FB Setpoint (mV)", y=3.2767) -> (x*y=w2028:dbl)
        n1404 = Multiply(x="Blue Intensity % (FB OFF)", y=655.35) -> (x*y=w2031:dbl)
        n1405 = To Unsigned Word Integer(number=w2031) -> (unsigned 16bit integer=w2030:u16)
        n1406 = local read "Laser interlacing mode"() -> (w2026:enum32{"Laser ON", "Laser OFF", "Interlace"})
        n1407 = Unbundle By Name("Blue FB Gains") -> ("proportional gain (Kc)"=w2023:i16, "integral gain (Kc*Ts/Ti)"=w2022:i16, "derivative gain (Kc*Td/Ts)"=w2021:i16)
        n1408 = local read "Blue Laser ON"() -> (w2015:bool)
        n1409 = Equal?(x=w2026, y=enum32{"Laser ON", "Laser OFF", "Interlace"}."Interlace") -> (x = y?=w2024:bool)
        n1410 = Compound Arithmetic op=AND(w2024, "Blue FB On/Off", w2015) -> (w2027:bool)
        n1411 = xnode "Read/Write Control"("FPGA VI Reference In"=w2035, "error in"=w2034, "Blue FB Setpoint"=w2028, "Blue FB On/Off"=w2027, "BI Current Out"=w2030, "Blue current ON count adj (AO)"="Blue int AO ON count adjust", "P5"=w2023, "I5"=w2022, "D5"=w2021) -> ("error out"=w2033:errorcluster)  [unwired: 1 out]
      }
      event "Red FB Setpoint (mV)", "Red FB Gains", "Red FB On/Off", "Red Intensity % (FB OFF)", "Red int current ON count adj": Value Change {
        n1412 = event-data() -> ()  [unwired: 7 out]
        n1413 = local read "Red FB Setpoint (mV)"() -> (w2047:dbl)
        n1414 = Multiply(x=w2047, y=3.2767) -> (x*y=w2046:dbl)
        n1415 = local read "Red Intensity % (FB OFF)"() -> (w2036:dbl)
        n1416 = Multiply(x=w2036, y=655.35) -> (x*y=w2050:dbl)
        n1417 = To Unsigned Word Integer(number=w2050) -> (unsigned 16bit integer=w2049:u16)
        n1418 = local read "Red int current ON count adj"() -> (w2052:u16)
        n1419 = local read "Laser interlacing mode"() -> (w2043:enum32{"Laser ON", "Laser OFF", "Interlace"})
        n1420 = local read "Red FB Gains"() -> (w2040:T9)
        n1421 = local read "Red Laser ON"() -> (w2044:bool)
        n1422 = local read "Red FB On/Off"() -> (w2053:bool)
        n1423 = Equal?(x=w2043, y=enum32{"Laser ON", "Laser OFF", "Interlace"}."Interlace") -> (x = y?=w2041:bool)
        n1424 = Unbundle By Name(w2040) -> ("proportional gain (Kc)"=w2039:i16, "integral gain (Kc*Ts/Ti)"=w2038:i16, "derivative gain (Kc*Td/Ts)"=w2037:i16)
        n1425 = Compound Arithmetic op=AND(w2041, w2053, w2044) -> (w2045:bool)
        n1426 = xnode "Read/Write Control"("FPGA VI Reference In"=w2056, "error in"=w2055, "Red FB Setpoint"=w2046, "Red FB On/Off"=w2045, "RI Current Out"=w2049, "Red int current ON count adj"=w2052, "P4"=w2039, "I4"=w2038, "D4"=w2037) -> ("error out"=w2054:errorcluster)  [unwired: 1 out]
      }
      event "+ phase (APD 1 Gate)", "- phase (APD 1 Gate)", "+ phase (APD 2 Gate)", "- phase (APD 2 Gate)", "+ phase (APD 3 Gate)", "- phase (APD 3 Gate)", "+ phase (APD Acq)", "- phase (APD Acq)": Value Change {
        n1427 = event-data() -> ()  [unwired: 7 out]
        n1428 = local read "Phase Adj. (APD 1 Gate)"() -> (w2076:i16)
        n1429 = Or(x="- phase (APD 1 Gate)", y="+ phase (APD 1 Gate)") -> (x .or. y?=w2078:bool)
        n1430 = Negate(x=w2076) -> (-x=w2083:i16)
        n1431 = Select(t=w2083, s="+ phase (APD 1 Gate)", f=w2076) -> (s? t:f=w2082:i16)
        n1432 = local read "Phase Adj. (APD 2 Gate)"() -> (w2073:i16)
        n1433 = Or(x="- phase (APD 2 Gate)", y="+ phase (APD 2 Gate)") -> (x .or. y?=w2071:bool)
        n1434 = Negate(x=w2073) -> (-x=w2075:i16)
        n1435 = Select(t=w2075, s="+ phase (APD 2 Gate)", f=w2073) -> (s? t:f=w2072:i16)
        n1436 = Negate(x="Phase Adj. (APD 3 Gate)") -> (-x=w2070:i16)
        n1437 = Or(x="- phase (APD 3 Gate)", y="+ phase (APD 3 Gate)") -> (x .or. y?=w2066:bool)
        n1438 = Select(t=w2070, s="+ phase (APD 3 Gate)", f="Phase Adj. (APD 3 Gate)") -> (s? t:f=w2067:i16)
        n1439 = local read "Phase Adj. (APD Acq)"() -> (w2064:i16)
        n1440 = Or(x="- phase (APD Acq)", y="+ phase (APD Acq)") -> (x .or. y?=w2062:bool)
        n1441 = Negate(x=w2064) -> (-x=w2065:i16)
        n1442 = Select(t=w2065, s="+ phase (APD Acq)", f=w2064) -> (s? t:f=w2063:i16)
        n1443 = xnode "Read/Write Control"("FPGA VI Reference In"=w2085, "error in"=w2084, "Phase count adjustment (APD 1 Gate)"=w2082, "Phase count adjustment (APD 2 Gate)"=w2072, "Phase count adjustment (APD 3 Gate)"=w2067, "Phase Count Adjustment (APD Acq)"=w2063) -> ("FPGA VI Reference Out"=w2080:T19, "error out"=w2081:errorcluster)
        n1444 = xnode "Read/Write Control"("FPGA VI Reference In"=w2080, "error in"=w2081, "+ phase (APD 1 Gate)"=w2078, "+ phase (APD 2 Gate)"=w2071, "+ phase (APD 3 Gate)"=w2066, "+ phase (APD Acq)"=w2062) -> ("error out"=w2079:errorcluster)  [unwired: 1 out]
      }
      event "Invert APD Gate", "APD Gate ON Count", "APD Gate OFF Count", "APD Gate", "APD Integration Time (s)", "APD AO Scale Factor", "Duty Frequency (ON 1/N cycles)", "Interlace ON count", "Interlace OFF count": Value Change {
        n1445 = event-data() -> ()  [unwired: 7 out]
        n1446 = Add(x="Interlace ON count", y="Interlace OFF count") -> (x+y=w2091:u16)
        n1447 = Add(x="APD Gate ON Count", y="APD Gate OFF Count") -> (x+y=w2102:u16)
        n1448 = Multiply(x="Duty Frequency (ON 1/N cycles)", y=w2091) -> (x*y=w2087:u16)
        "Green AI Count" <- w2087
        "Red AI Count" <- w2087
        "Blue AI Count" <- w2087
        n1449 = Subtract(x=w2087, y="Interlace ON count") -> (x-y=w2090:u16)
        n1450 = Multiply(x=w2102, y="Duty Frequency (ON 1/N cycles)") -> (x*y=w2101:u16)
        n1451 = Subtract(x=w2101, y="APD Gate ON Count") -> (x-y=w2100:u16)
        n1452 = local read "DMA Update Period (s)"() -> (w2103:dbl)
        n1453 = Multiply(x="APD Integration Time (s)", y=40000000.0) -> (x*y=w2107:dbl)
        n1454 = Reciprocal(x="APD Integration Time (s)") -> (1/x=→"APD Acq Rate (Hz)":dbl)
        n1455 = To Unsigned Long Integer(number=w2107) -> (unsigned 32bit integer=w2093:u32)
        "APD Int. Count" <- w2093
        n1456 = local read "Number of APDs"() -> (w2086:u8)
        n1457 = Divide(x=w2103, y="APD Integration Time (s)") -> (x/y=w2105:dbl)
        n1458 = Multiply(x=w2086, y=w2105) -> (x*y=w2104:dbl)
        n1459 = local write "APD Samples/FIFO Acq."(w2105) -> ()
        n1460 = local write "APD Elements/DMA read"(w2104) -> ()
        n1461 = xnode "Read/Write Control"("FPGA VI Reference In"=w2111, "error in"=w2110, "Invert APD Gate"="Invert APD Gate", "APD Gate ON Count"="APD Gate ON Count", "APD Gate OFF Count"=w2100, "APD Acq Rate Count"=w2093, "APD Gate Operating Mode"="APD Gate", "APD AO scale factor"="APD AO Scale Factor", "Green interlace ON count"="Interlace ON count", "Green interlace OFF count"=w2090, "Green interlace ON count 2"="Interlace ON count", "Green interlace OFF count 2"=w2090, "Green FB Count"=w2087, "Red interlace ON count"="Interlace ON count", "Red interlace OFF count"="Interlace OFF count", "Red FB Count"=w2087, "Red interlace ON count 2"="Interlace ON count", "Red interlace OFF count 2"="Interlace OFF count", "Blue ON count (AO)"="Interlace ON count", "Blue OFF count (AO)"="Interlace OFF count", "Blue interlace OFF count (D)"="Interlace OFF count", "Blue interlace ON count (D)"="Interlace ON count", "Blue Int Count"=w2087) -> ("error out"=w2109:errorcluster)  [unwired: 1 out]
      }
      event "Neg. TTrig FPGA": Value Change {
        n1462 = event-data() -> ()  [unwired: 7 out]
        n1463 = xnode "Read/Write Control"("FPGA VI Reference In"=w2114, "error in"=w2113, "TTrig Negate Pos"="Neg. TTrig FPGA") -> ()  [unwired: 2 out]
      }
      event "Test ttrig": Value Change {
        n1464 = event-data() -> ()  [unwired: 7 out]
        n1465 = xnode "Read/Write Control"("FPGA VI Reference In"=w2118, "error in"=w2117, "TTrig?"=TRUE) -> ("error out"=w2116:errorcluster)  [unwired: 1 out]
      }
      event "Number of F/B Scans (AOD)", "Scan Speed (nm/s)", "Scan BD", "Initial delta (MHz)", "Step Size (nm)", "Scan Range (nm)": Value Change {
        w2181 = 123.0  # AOM cal (nm/MHz)
        n1466 = event-data() -> ()  [unwired: 7 out]
        n1467 = local read "BD 1 Frequency 1 (MHz)"() -> (w2164:dbl)
        n1468 = local read "AOM X Cal (nm/MHz)"() -> (w2156:dbl)
        n1469 = local read "X RF Frequency Limits (MHz)"() -> (w2168:T16)
        n1470 = local read "Y RF Frequency Limits (MHz)"() -> (w2165:T16)
        n1471 = local read "BD 2 Frequency 1 (MHz)"() -> (w2170:dbl)
        n1472 = Negate(x="Scan Range (nm)") -> (-x=w2134:dbl)
        n1473 = Divide(x=w2134, y=w2156) -> (x/y=w2138:dbl)
        n1474 = Select(t=w2168, s="Scan BD", f=w2165) -> (s? t:f=w2167:T16)
        n1475 = Select(t=w2164, s="Scan BD", f=w2170) -> (s? t:f=w2169:dbl)
        n1476 = Unbundle By Name(w2167) -> ("Maximum"=w2176:dbl, "Minimum"=w2175:dbl)
        n1477 = Add(x=w2138, y=w2169) -> (x+y=w2173:dbl)
        n1478 = Divide(x=w2134, y="Step Size (nm)") -> (x/y=w2153:dbl)
        n1479 = Divide(x="Step Size (nm)", y=w2156) -> (x/y=w2162:dbl)
        n1480 = Absolute Value(x=w2153) -> (abs(x)=w2137:dbl)
        n1481 = Sign(1:w2134) -> (0:w2135:dbl)
        n1482 = In Range and Coerce(upper limit=w2176, x=w2173, lower limit=w2175) -> (coerced(x)=w2172:dbl, In Range?=w2174:bool)
        n1483 = To Unsigned Quad Integer(1:w2137) -> (0:w2152:u64)
        "Scan steps (AOD)" <- w2152
        n1484 = call "IR AOM freq to word.vi"("Frequency In (MHz)"=w2162) -> ("Frequency Word Out (double)"=w2159:dbl)
        n1485 = Multiply(x=w2135, y=w2159) -> (x*y=w2136:dbl)
        n1486 = Subtract(x=w2173, y=w2172) -> (x-y=w2171:dbl)
        n1487 = To Quad Integer(1:w2136) -> (0:w2158:i64)
        "Incr. int (AOD)" <- w2158
        n1488 = Subtract(x=w2138, y=w2171) -> (x-y=w2157:dbl)
        "Scan Range (MHz)" <- w2157
        n1489 = Select(t=w2138, s=w2174, f=w2157) -> (s? t:f=w2177:dbl)
        n1490 = Multiply(x=w2157, y=w2156) -> (x*y=w2155:dbl)
        n1491 = Decrement(x=w2152) -> (x-1=w2205:u64)
        n1492 = Negate(x=w2155) -> (-x=w2151:dbl)
        n1493 = local write "Scan Range (nm)"(w2151) -> ()
        n1494 = Divide(x=w2177, y=w2205) -> (x/y=w2161:dbl)
        "Scan Increment (MHz)" <- w2161
        n1495 = call "IR AOM freq to word.vi"("Frequency In (MHz)"=w2161) -> ("Frequency Word Out (double)"=w2160:dbl)
        n1496 = Divide(x="Step Size (nm)", y="Scan Speed (nm/s)") -> (x/y=w2148:dbl)
        n1497 = To Quad Integer(1:w2160) -> ()  [unwired: 1 out]
        n1498 = local read "Number Interlace Sets"() -> (w2132:u8)
        n1499 = local read "AI Count (ticks)"() -> (w2133:u16)
        n1500 = local read "Total Counts (ticks)"() -> (w2131:u16)
        n1501 = local read "# Samples/trap"() -> (w2163:u32)
        n1502 = Multiply(x=w2133, y=w2132) -> (x*y=w2130:u16)
        n1503 = Divide(x=w2131, y=w2130) -> (x/y=w2129:dbl)
        n1504 = Select(t=w2164, s="Scan BD", f=w2170) -> (s? t:f=w2202:dbl)
        "Initial freq. (MHz)" <- w2202
        n1505 = Add(x=w2177, y=w2202) -> (x+y=→"Final freq. (MHz)":dbl)
        n1506 = Divide(x=w2131, y=40000000.0) -> (x/y=w2147:dbl)
        n1507 = Divide(x=w2148, y=w2147) -> (x/y=w2146:dbl)
        n1508 = To Unsigned Quad Integer(1:w2146) -> (0:w2121:u64)
        n1509 = Quotient & Remainder(x=w2121, y=u64 2) -> (x-y*floor(x/y)=w2125:u64)  [unwired: 1 out]
        n1510 = Equal?(x=w2125, y=u64 0) -> (x = y?=w2123:bool)
        n1511 = Decrement(x=w2121) -> (x-1=w2122:u64)
        n1512 = Select(t=w2121, s=w2123, f=w2122) -> (s? t:f=w2120:u64)
        "Cycles/step (AOD)" <- w2120
        n1513 = xnode "Read/Write Control"("FPGA VI Reference In"=w2213, "error in"=w2212, "Scan steps"=w2152, "Number of scans"="Number of F/B Scans (AOD)", "Cycles per step"=w2120, "Scan freq.  increment"=w2158, "Scan BD"="Scan BD") -> ("error out"=w2211:errorcluster)  [unwired: 1 out]
        n1514 = Multiply(x=w2152, y=w2120) -> (x*y=w2206:u64)
        n1515 = Multiply(x=w2206, y=u64 2) -> (x*y=w2128:u64)
        n1516 = Multiply(x=w2129, y=w2128) -> (x*y=w2127:dbl)
        "Data points/scan (f/b)" <- w2127
        n1517 = Multiply(x=w2127, y="Number of F/B Scans (AOD)") -> (x*y=w2209:dbl)
        "Data points/scans" <- w2209
        n1518 = Divide(x=w2209, y=w2163) -> (x/y=→"N sets should be saved":dbl)
        n1519 = Multiply(x=w2206, y=w2147) -> (x*y=w2145:dbl)
        "Time/Scan (s) (AOD)" <- w2145
        n1520 = Select(t=w2177, s="Scan BD", f=0.0) -> (s? t:f=w2203:dbl)
        n1521 = Select(t=0.0, s="Scan BD", f=w2177) -> (s? t:f=w2199:dbl)
        n1522 = local read "BD 2 Frequency 2 (MHz)"() -> (w2195:dbl)
        n1523 = local read "BD 1 Frequency 2 (MHz)"() -> (w2198:dbl)
        n1524 = Add(x=w2199, y=w2170) -> (x+y=w2196:dbl)
        n1525 = Add(x=w2164, y=w2203) -> (x+y=w2197:dbl)
        n1526 = Multiply(x=w2145, y=2.0) -> (x*y=w2144:dbl)
        n1527 = Multiply(x=w2144, y="Number of F/B Scans (AOD)") -> (x*y=w2141:dbl)
        n1528 = Divide(x=w2141, y=60.0) -> (x/y=→"Time to Finish All (min)":dbl)
        n1529 = Add(x="Trap 2 Bead Size (nm)", y="Trap 1 Bead Size (nm)") -> (x+y=w2185:dbl)
        n1530 = Divide(x=w2185, y=2.0) -> (x/y=w2179:dbl)
        n1531 = local read "Initial delta (MHz)"() -> (w2182:dbl)
        n1532 = Subtract(x=w2196, y=w2195) -> (x-y=w2193:dbl)
        n1533 = Subtract(x=w2197, y=w2198) -> (x-y=w2194:dbl)
        n1534 = Square(x=w2193) -> (x^2=w2192:dbl)
        n1535 = Square(x=w2194) -> (x^2=w2191:dbl)
        n1536 = Add(x=w2191, y=w2192) -> (x+y=w2190:dbl)
        n1537 = Square Root(x=w2190) -> (sqrt(x)=w2189:dbl)
        "Final delta (MHz)" <- w2189
        n1538 = Multiply(x=w2181, y=w2189) -> (x*y=w2188:dbl)
        n1539 = Multiply(x=w2182, y=w2181) -> (x*y=w2180:dbl)
        n1540 = Subtract(x=w2180, y=w2179) -> (x-y=→"Initial sep (nm)":dbl)
        n1541 = Subtract(x=w2188, y=w2179) -> (x-y=→"Final sep (nm)":dbl)
      }
      event "Freq or Amp switch first", "Swap F1 and F2", "Freq switch delay", "Amp switch delay": Value Change {
        n1542 = event-data() -> ()  [unwired: 7 out]
        n1543 = local read "Amp switch delay"() -> (w2214:u16)
        n1544 = local read "Swap F1 and F2"() -> (w2215:bool)
        n1545 = xnode "Read/Write Control"("FPGA VI Reference In"=w2218, "error in"=w2217, "Swap F1 and F2"=w2215, "Amp switch delay"=w2214) -> ("error out"=w2216:errorcluster)  [unwired: 1 out]
      }
      event "Scan steps (MCL)", "Number of scans (MCL)", "Scan Range (V)\n(of steps)", "2D or 1D Scan", "N APD Samp/step", "Fast Scan Dir", "Continuous MCL Scanning", "Scan lines (y)": Value Change {
        w2220 = 32767.0 ("y")
        n1546 = event-data() -> ()  [unwired: 7 out]
        n1547 = Select(t="Scan lines (y)", s="2D or 1D Scan", f="Number of scans (MCL)") -> (s? t:f=w2225:u64)
        n1548 = Decrement(x="Scan steps (MCL)") -> (x-1=w2241:u64)
        n1549 = Divide(x="Scan Range (V)\n(of steps)", y=w2241) -> (x/y=w2240:dbl)
        "Desired Scan Incr (V)" <- w2240
        n1550 = local read "APD Integration Time (s)"() -> (w2233:dbl)
        n1551 = Multiply(x=w2240, y=w2220) -> (x*y=w2249:dbl)
        n1552 = Divide(x=w2249, y=10.0) -> (x/y=w2239:dbl)
        "Desired incr (int)" <- w2239
        n1553 = local read "Update Count (MCL)"() -> (w2245:u32)
        n1554 = Round Toward -Infinity(1:w2239) -> (0:w2248:dbl)
        n1555 = To Word Integer(number=w2248) -> (16bit integer=w2223:i16)
        "Actual Incr. int (MCL)" <- w2223
        n1556 = Multiply(x=w2233, y=40000000.0) -> (x*y=w2246:dbl)